vi "Modelo planta H2_V2.vi"() -> ()   [LabVIEW 2022 SP3]
uses:
  <vilib>/Utility/file.llb/Read Delimited Spreadsheet (DBL).vi
panel:
  out "Compresor":bool
  out "stop 2":bool
  in  "stop":bool
  out "masa total P g":dbl format="%#.1f"
  out "H2 generado dia":dbl format="%#.1f"
  in  "Energía acum H2 verde inicio":dbl=527.0
  out "Energía solar diaría":dbl format="%#.1f"
  in  "Producción Solar total inicio":dbl=3421.0
  in  "H2 generado inicio":dbl=202.8
  out "g H2 consumidos por la FC":dbl
  out "H2 consumido en el lab":dbl=182.6 format="%#.1f"
  out "Numeric 9":dbl format="%#.1f"
  out "Energía acum H2 verde":dbl format="%#.1f"
  out "Producción Solar toral":dbl format="%#.1f"
  out "H2 generado Total":dbl format="%#.1f"
  in  "Forzar Comp":bool
  in  "Pot FC":dbl min=0.0 max=5.0 step=0.5
  in  "Forzar FC":bool
  out "Numeric 4":dbl format="%#.4g"
  out "Potència inversor solar":dbl(graph)
  out "masa total G g":dbl format="%#.0f"
  out "P alta":dbl format="%#.1f"
  out "P baja":dbl format="%#.1f"
  out "Numeric 3":dbl format="%#.4g"
  out "Producción FC":dbl format="%#_2g"
  out "Numeric":dbl format="%#.2f"
  out "Pressió tanc baixa":dbl(graph)
  out "Energia solar no utilitzada":dbl(graph)
  out "Producció d'hidrogen":dbl(graph)
  out "g comprimidos":dbl
  in  "Caudal compresor":dbl
  out "P tanq alta (barg)":dbl(graph)
  out "P tanq baja (barg)":dbl(graph)
  in  "Presión ini Tanq baba":dbl=28.0
  in  "Presión ini Tanq alta":dbl=220.0
  in  "Nº electro":u8 max=6 step=1
  in  "Forzar":bool
  out "Energía Solar no usada (kWh)":dbl(graph)
  out "H2 acumulado diario (g)":dbl(graph)
  out "Producción instalan (g/s)":dbl(graph)
  out "Electroli ON":dbl(graph)
  out "Potencia Consumo electroli instan. (kW)":dbl(graph)
  out "Producción diaria (g)":dbl
  out "Producción instalan (g/s)":dbl
  out "Electroli ON":dbl
  in  "Soleado/Nublado":bool=TRUE
  out "Minuto":i32
  in  "tiempo ejecución":u32=1000
  out "Potencia Solar Instanta (kW)":dbl(graph)
  out "Nublado":dbl[](array[numeric])
  out "Soleado":dbl[](array[numeric])
  out "Minuto":i32
  out "min":i32
  out "Hora":i32
  out "current time":timestamp format="%<%H:%M\n%x>T"
  in  "milliseconds to wait":u32=250
  out "Nublado":dbl[](graph)
  out "Soleado":dbl[](graph)
  # "H2 baixa pressió"
  # "H2 alta pressió"
  # "kW"
  # "barg"
  # "Tanc baixa pressió"
  # "Tanc alta pressió"
  # "Electrolizador"
  # "Compressor"
  # "g/s"
  # "barg"
  # "Solar"
  # "Fuel Cell"
  # "kW"
  # "kW"
  # "g"
  # "g"
  # "Elect ON"
  # "Xarxa electrica"
  # "-"
  # "+"
  # "kW de xarxa"
  # "Producció total d'hidrogen"
  # "Producció d'hidrogen diària"
  # "g"
  # "kg"
  # "Producció total d'energia solar"
  # "Energia solar produïda diària"
  # "kWh"
  # "kWh"
  # "Energia acumulada per H2 verd"
  # "Consum de H2 Lab diari"
  # "g"
  # "kWh"
  # "g"
  # "bar"
  # "bar"
  # "kg"
  # "kWh"
  # "kWh"
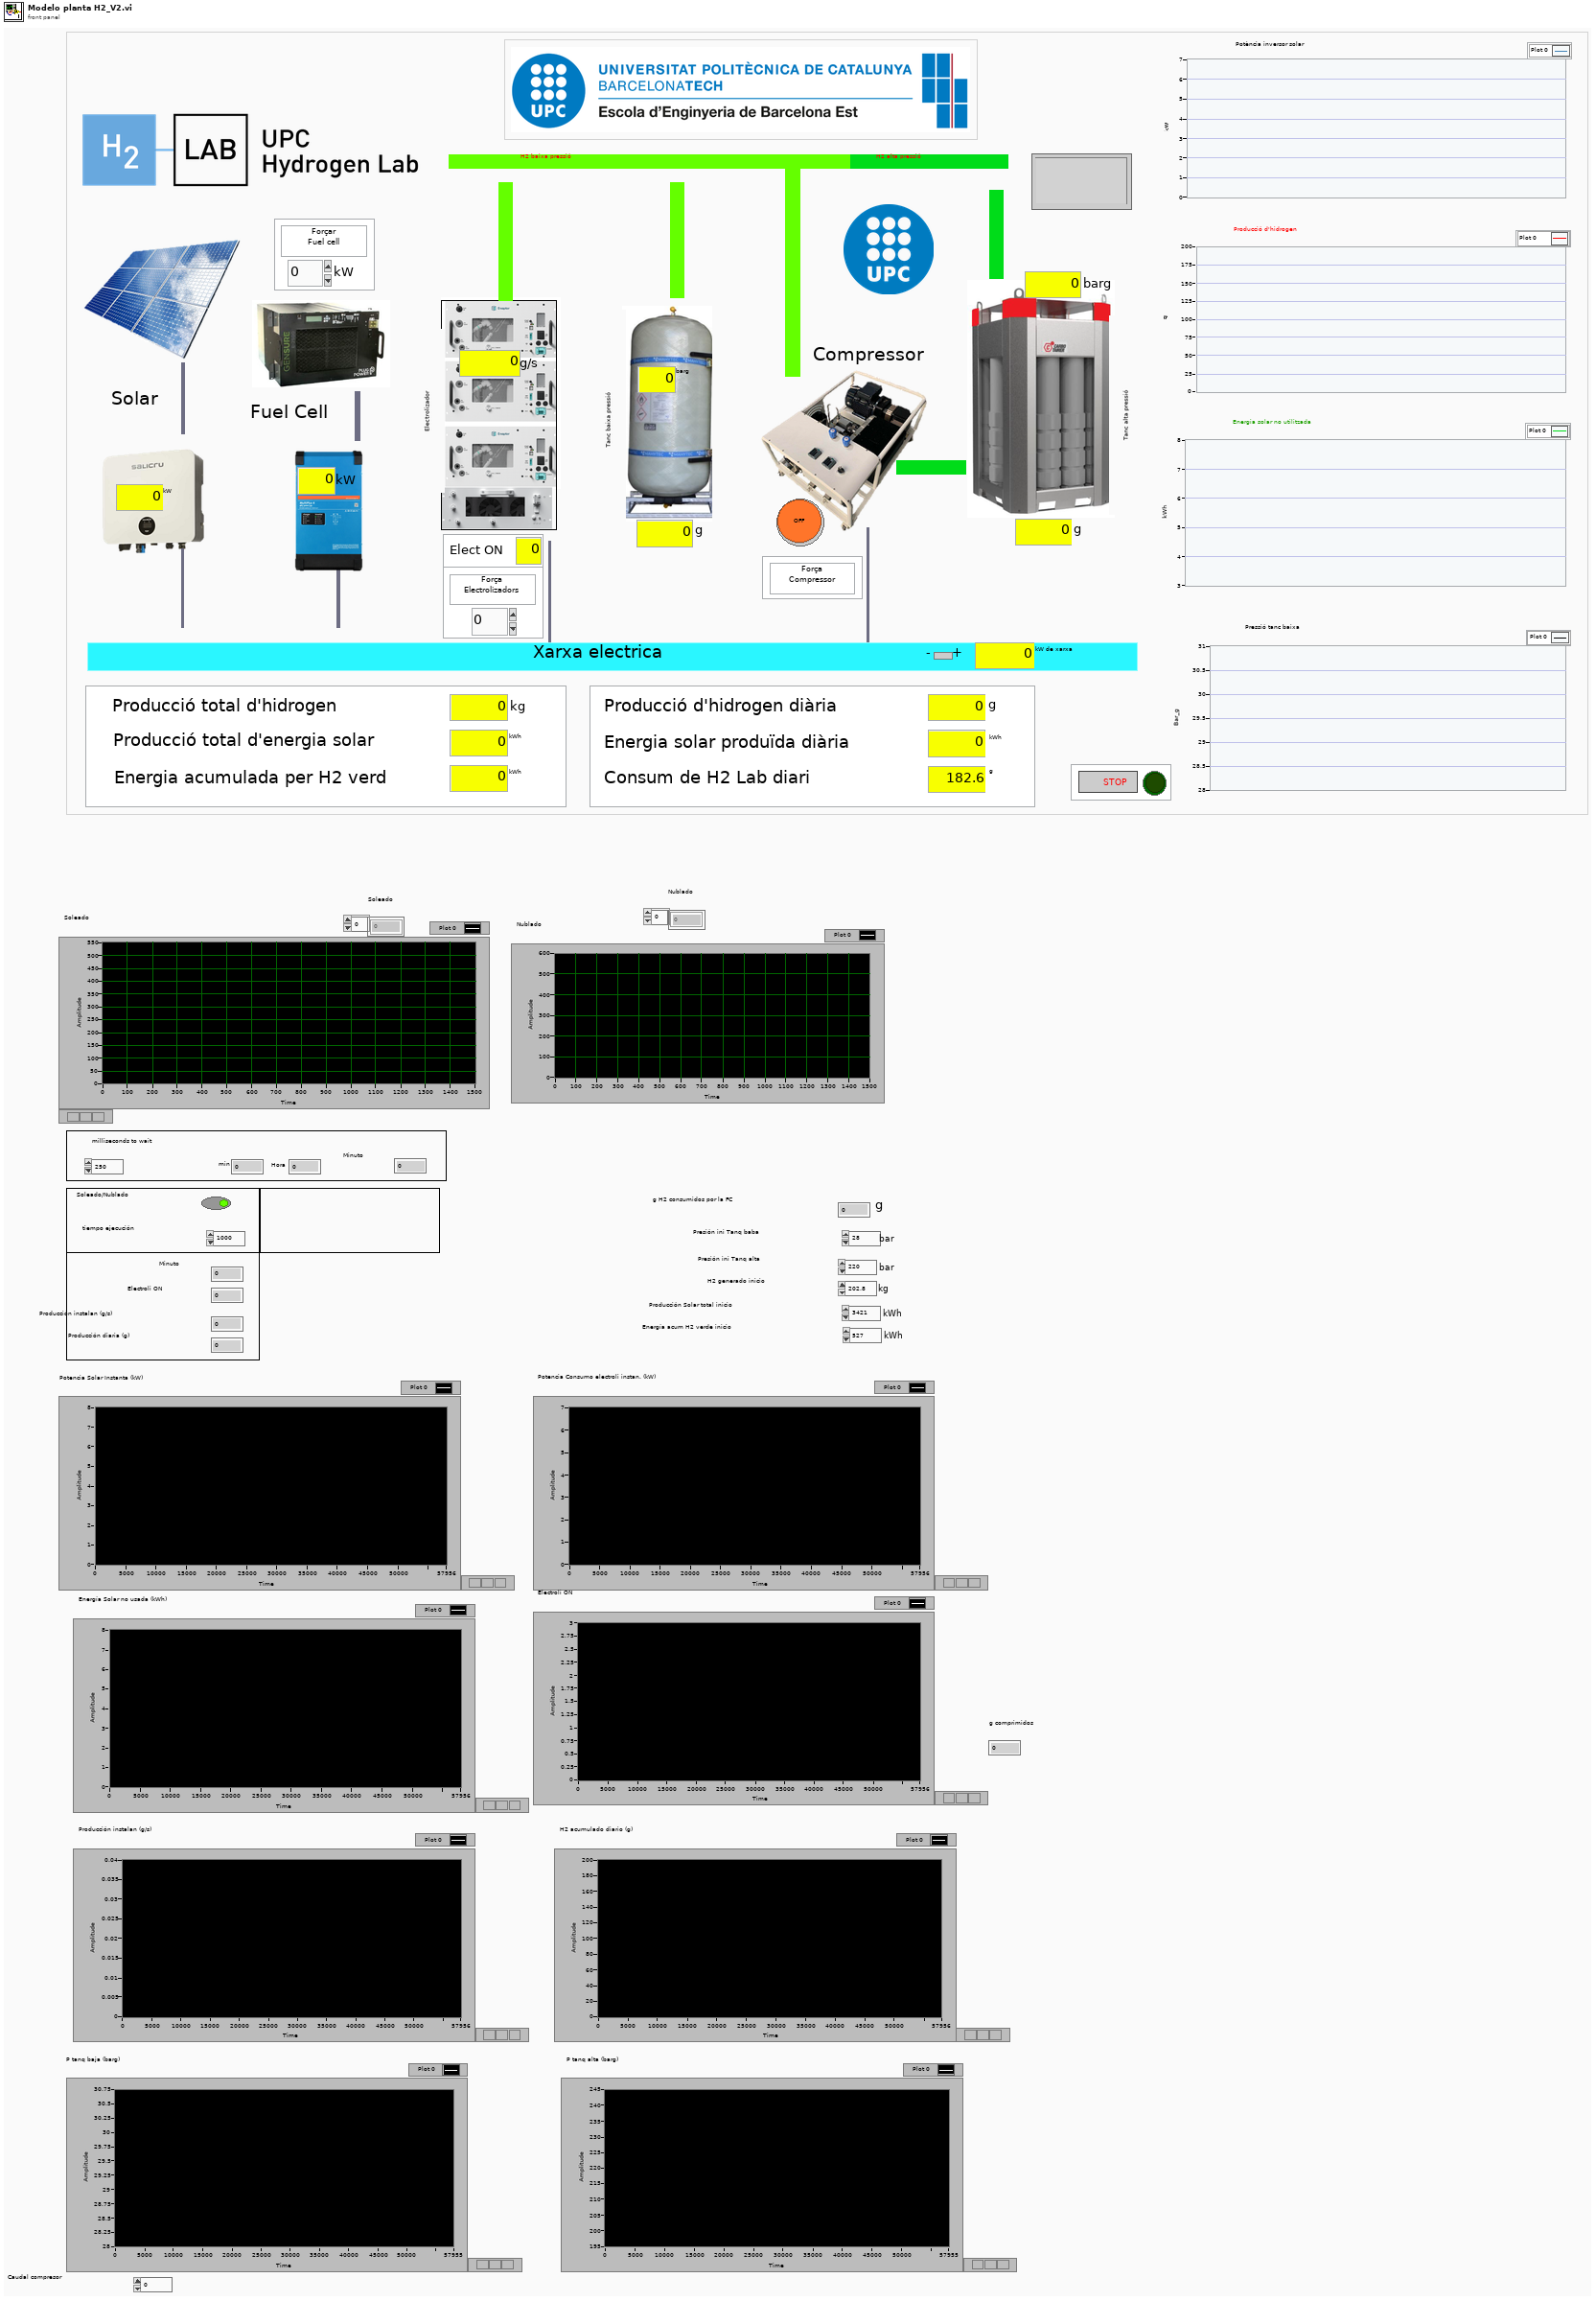
[diagram p1: front panel]
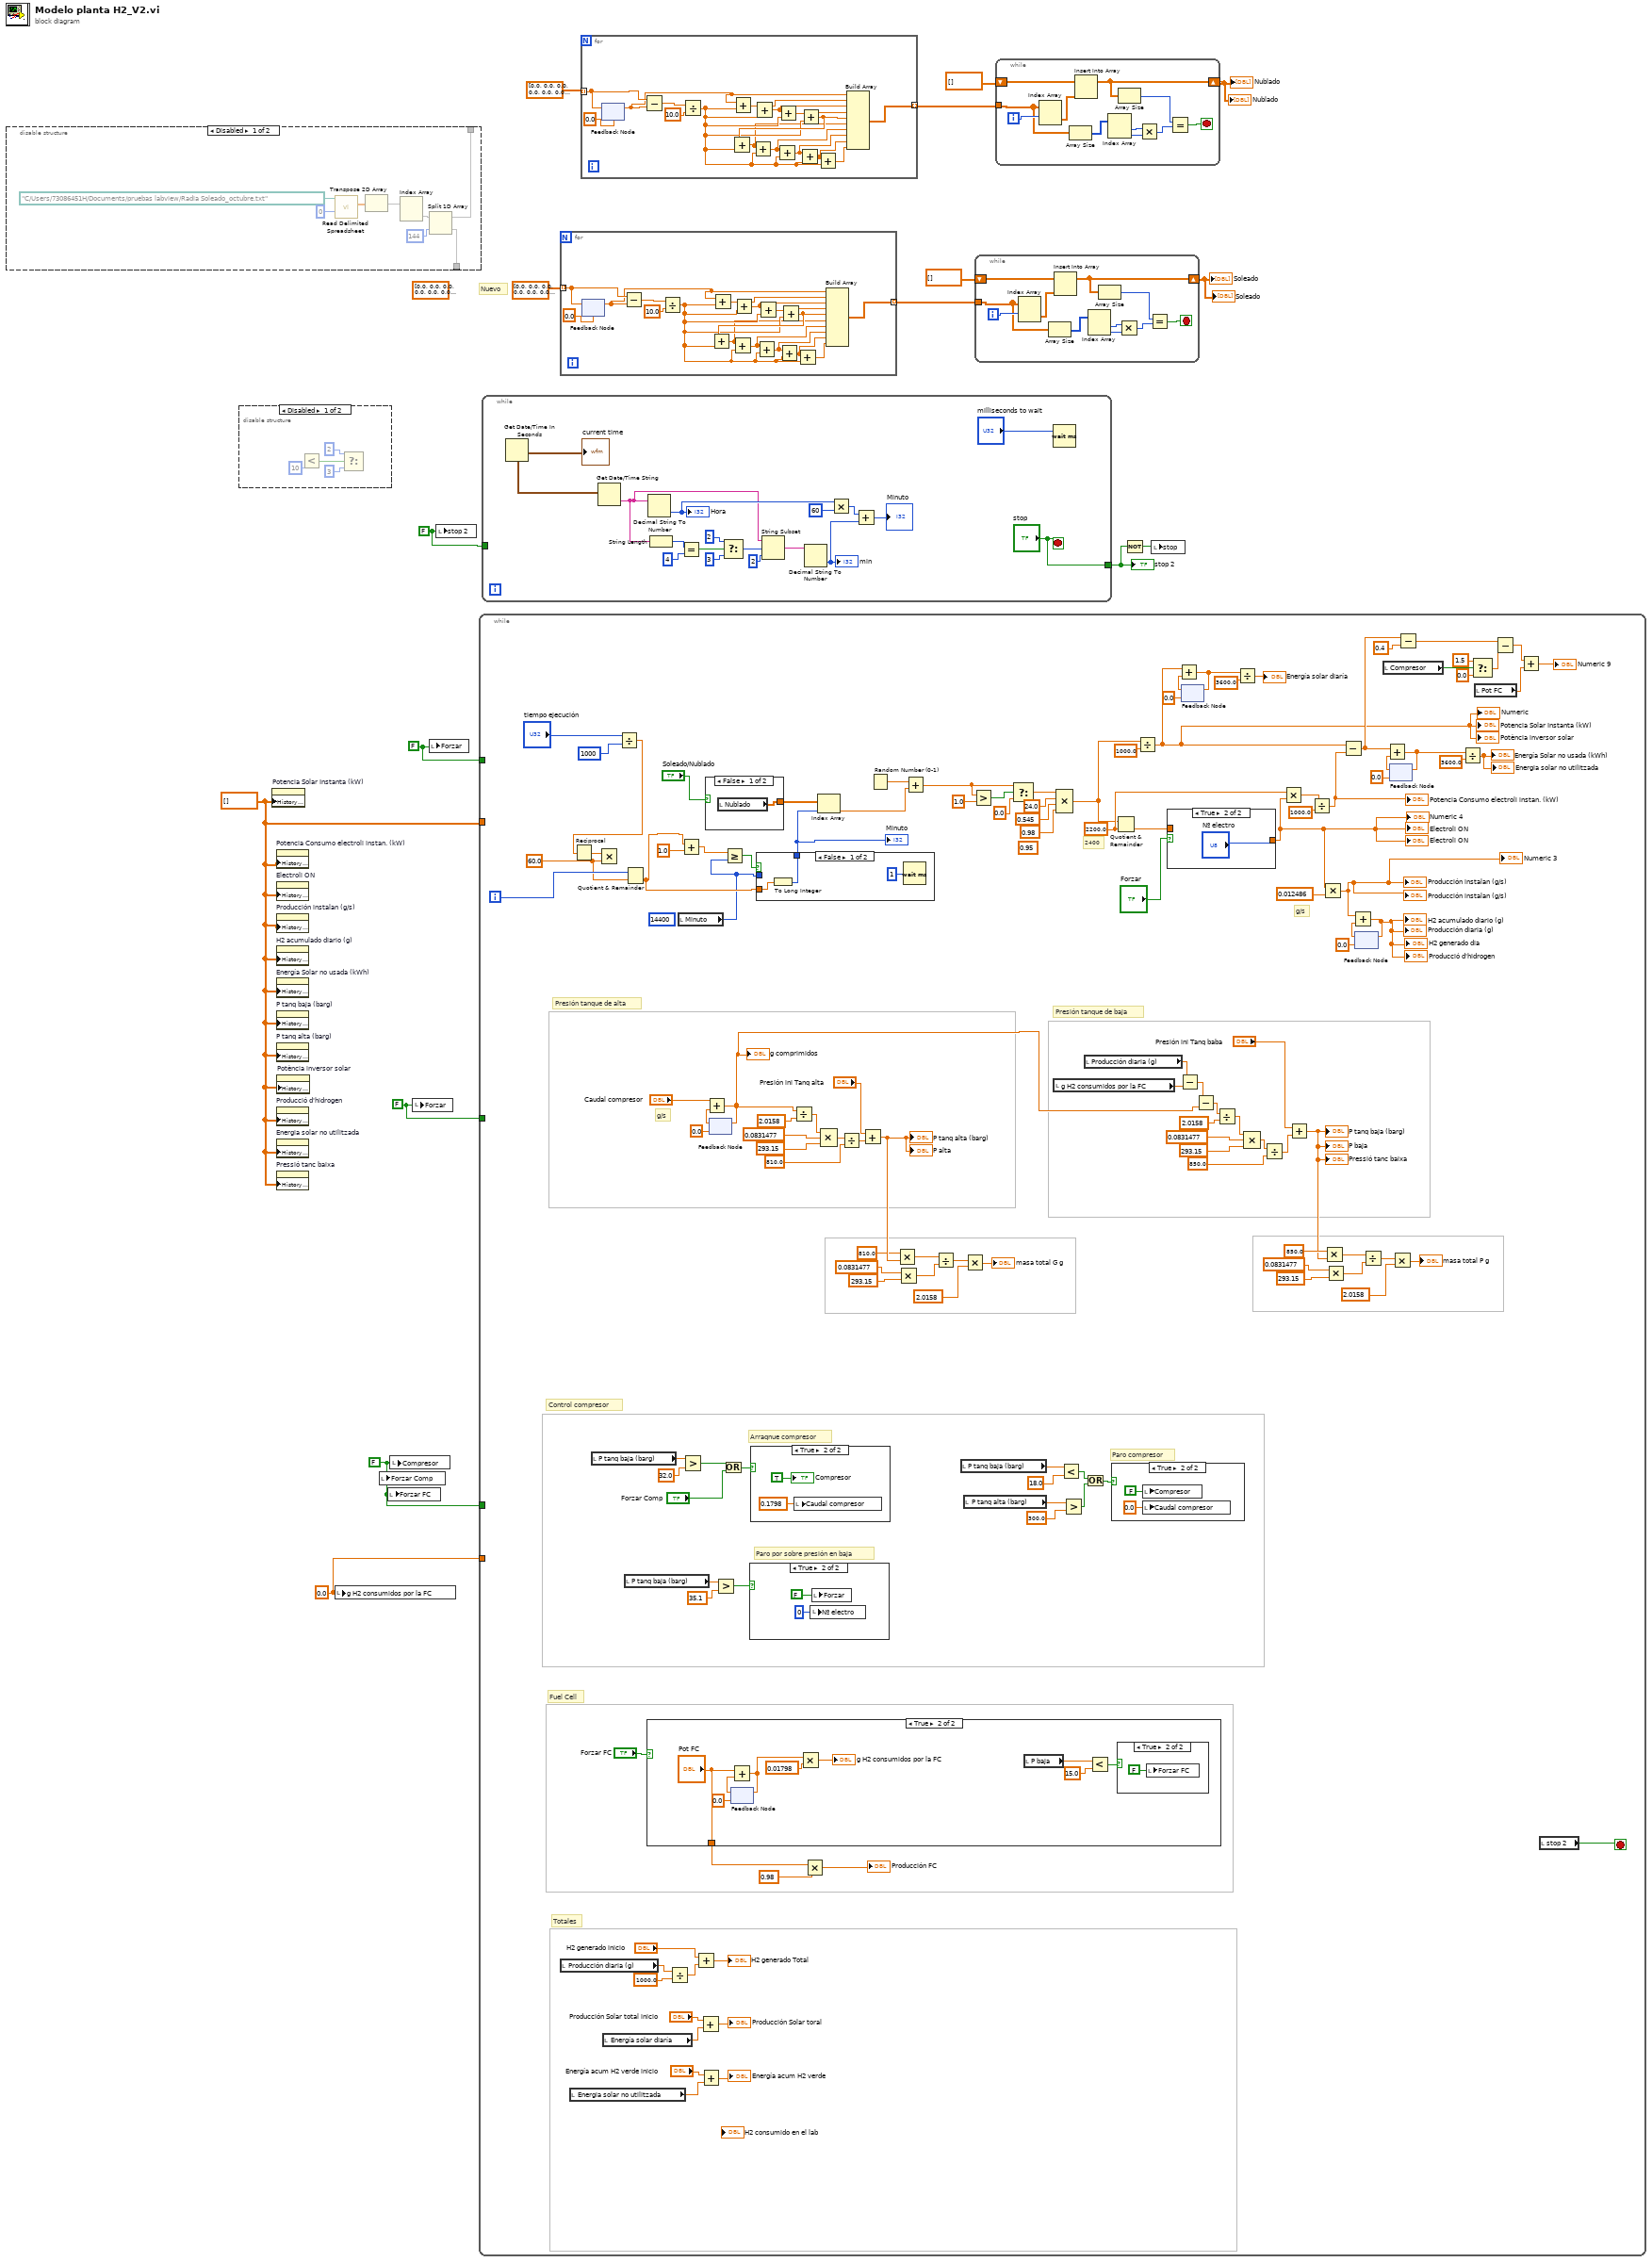
[diagram p0: block diagram]
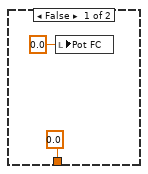
[diagram p4: hidden frame]
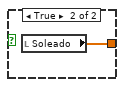
[diagram p10: hidden frame]
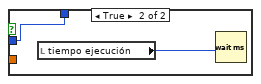
[diagram p11: hidden frame]
diagram:
  w1 = 0.0 ("g H2 consumidos por la FC")
  w3 = FALSE ("stop 2")
  w2 = FALSE ("Compresor")
  (unwired) dbl[] [0.0, 0.0, 0.0, 0.0, 0.0, 0.0, 0.0, 0.0, 0.0, 0.0, 0.0, 0.0, 0.0, 0.0, 0.0, 0.0, 0.0, 0.0, 0.0, 0.0, 0.0, 0.0, 0.0, 0.0, 0.0, 0.0, 0.0, 0.0, 0.0, 0.0, 0.0, 0.0, 0.0, 0.0, 0.0, 0.0, 0.0, 0.0, 0.0, 0.0, 0.0, 0.0, 0.0, 0.0, 0.0, 0.0, 0.0, 20.0, 56.927, 86.927, 116.927, 146.927, 176.927, 206.927, 236.927, 266.927, 296.927, 328.503, 349.407, 367.451, 386.007, 402.123, 418.893, 433.628, 449.442, 458.386, 484.691, 483.049, 496.591, 507.51, 517.195, 522.329, 530.995, 539.123, 538.419, 539.353, 541.627, 542.358, 542.375, 538.101, 543.836, 544.81, 539.48, 533.752, 526.738, 517.297, 506.831, 496.206, 486.59, 477.59, 460.949, 445.951, 431.313, 417.619, 400.78, 383.627, 364.764, 346.383, 329.104, 311.132, 291.528, 271.047, 249.886, 227.664, 206.918, 185.245, 162.013, 141.586, 121.314, 100.961, 79.259, 58.513, 35.892, 22.622, 4.309, 0.0, 0.0, 0.0, 0.0, 0.0, 0.0, 0.0, 0.0, 0.0, 0.0, 0.0, 0.0, 0.0, 0.0, 0.0, 0.0, 0.0, 0.0, 0.0, 0.0, 0.0, 0.0, 0.0, 0.0, 0.0, 0.0, 0.0, 0.0, 0.0] ("first subarray 2")
  w7 = FALSE ("Manual")
  w5 = dbl[] [] ("History Data")
  w9 = FALSE ("stop 2")
  # "Nuevo"
  n1 = disable-structure shown="Disabled" {
    disable-tunnel: [w18 _] -> _
    disable-tunnel: [w17 _] -> _
    frame Disabled {
      n2 = call-poly <vilib>:"Read Delimited Spreadsheet.vi"("file path (dialog if empty)"=path "C:/Users/73086451H/Documents/pruebas labview/Radia Soleado_octubre.txt", "start of read offset (chars.:0)"=0) -> ("all rows"=w23:dbl[][])  [unwired: 8 in, 5 out]
      n3 = Transpose 2D Array(2D array=w23) -> (transposed array=w22:dbl[][])
      n4 = Index Array(array=w22) -> (element=w20:dbl[])  [unwired: 2 in]
      n5 = Split 1D Array(array=w20, index=144) -> (first subarray=w18:dbl[], second subarray=w17:dbl[])
    }
    frame Enabled {
    }
  }
  n6 = disable-structure shown="Disabled" {
    frame Disabled {
      n7 = Less?(y=10) -> (x=w27:i32, x < y?=w29:bool)
      n8 = Select(t=2 ("offset (0)"), s=w29, f=3 ("offset (0)")) -> ()  [unwired: 1 out]
    }
    frame Enabled {
    }
  }
  n9 = property on="Potencia Solar Instanta (kW)" class="WFChart (strict)"("History Data"=w5) -> ()  [unwired: 2 in, 2 out]
  n10 = property on="Potencia Consumo electroli instan. (kW)" class="WFChart (strict)"("History Data"=w5) -> ()  [unwired: 2 in, 2 out]
  n11 = property on="Electroli ON" class="WFChart (strict)"("History Data"=w5) -> ()  [unwired: 2 in, 2 out]
  n12 = property on="Producción instalan (g/s)" class="WFChart (strict)"("History Data"=w5) -> ()  [unwired: 2 in, 2 out]
  n13 = property on="H2 acumulado diario (g)" class="WFChart (strict)"("History Data"=w5) -> ()  [unwired: 2 in, 2 out]
  n14 = property on="Energía Solar no usada (kWh)" class="WFChart (strict)"("History Data"=w5) -> ()  [unwired: 2 in, 2 out]
  n15 = property on="P tanq baja (barg)" class="WFChart (strict)"("History Data"=w5) -> ()  [unwired: 2 in, 2 out]
  n16 = property on="P tanq alta (barg)" class="WFChart (strict)"("History Data"=w5) -> ()  [unwired: 2 in, 2 out]
  n17 = property on="Producció d'hidrogen" class="WFChart (strict)"("History Data"=w5) -> ()  [unwired: 2 in, 2 out]
  n18 = property on="Energia solar no utilitzada" class="WFChart (strict)"("History Data"=w5) -> ()  [unwired: 2 in, 2 out]
  n19 = property on="Pressió tanc baixa" class="WFChart (strict)"("History Data"=w5) -> ()  [unwired: 2 in, 2 out]
  n20 = property on="Potència inversor solar" class="WFChart (strict)"("History Data"=w5) -> ()  [unwired: 2 in, 2 out]
  n21 = local write "g H2 consumidos por la FC"(w1) -> ()
  n22 = local write "Forzar Comp"(w2) -> ()
  n23 = local write "Forzar FC"(w2) -> ()
  n24 = local write "Compresor"(w2) -> ()
  n25 = local write "Forzar"(w7) -> ()
  n26 = local write "Forzar"(w3) -> ()
  n27 = local write "stop 2"(w9) -> ()
  n28 = while {
    tunnel: w5 -> [_]
    tunnel: w7 -> [_]
    tunnel: w2 -> [_]
    tunnel: w3 -> [_]
    tunnel: w1 -> [_]
    i -> [w161]
    stop <- w153 stop-if-true
    (unwired) 0.95 ("f")
    (unwired) 14400 ("Minuto")
    w134 = 2200.0 ("y")
    w139 = 60.0 ("y")
    # "Totales"
    # "Fuel Cell"
    # "Paro por sobre presión en baja"
    # "Paro compresor"
    # "Arraqnue compresor"
    # "g/s"
    # "Control compresor"
    # "Presión tanque de alta"
    # "Presión tanque de baja"
    # "g/s"
    # "2400"
    n29 = local read "Producción diaria (g)"() -> (w60:dbl)
    n30 = local read "Energia solar no utilitzada"() -> (w43:dbl)
    n31 = local read "P tanq baja (barg)"() -> (w116:dbl)
    n32 = local read "Energía solar diaría"() -> (w47:dbl)
    n33 = Divide(x="tiempo ejecución", y=u32 1000) -> (x/y=w150:dbl)
    n34 = Reciprocal(x=w150) -> (1/x=w144:dbl)
    n35 = Multiply(x=w144, y=w139) -> ()  [unwired: 1 out]
    n36 = local read "P tanq baja (barg)"() -> (w104:dbl)
    n37 = Quotient & Remainder(x=w161, y=w139) -> (floor(x/y)=w146:dbl)  [unwired: 1 out]
    n38 = case shown="True" "Forzar FC" {
      tunnel: [0.0 ("Pot FC") "Pot FC"] -> w39
      frame False {
        n39 = local write "Pot FC"(0.0 ("Pot FC")) -> ()
      }
      frame True {
        n40 = feedback #1(0.0) -> (w172:dbl)
        n41 = Add(x="Pot FC", y=w172) -> (x+y=w170:dbl)
        n42 = feedback-in #1(w170) -> ()
        n43 = Multiply(x=w170, y=0.01798) -> (x*y=→"g H2 consumidos por la FC":dbl)
        n44 = local read "P baja"() -> (w167:dbl)
        n45 = Less?(x=w167, y=15.0) -> (x < y?=w165:bool)
        n46 = case shown="True" w165 {
          frame False {
          }
          frame True {
            n47 = local write "Forzar FC"(FALSE ("Forzar FC")) -> ()
          }
        }
      }
    }
    n48 = Divide(x=w60, y=1000.0) -> (x/y=w58:dbl)
    n49 = local read "Minuto"() -> (w76:i32)
    n50 = Add(x=w146, y=1.0) -> (x+y=w147:dbl)
    n51 = Greater?(x=w116, y=32.0) -> (0:w70:bool)
    n52 = Add(x="H2 generado inicio", y=w58) -> (x+y=→"H2 generado Total":dbl)
    n53 = Add(x="Producción Solar total inicio", y=w47) -> (x+y=→"Producción Solar toral":dbl)
    n54 = Add(x="Energía acum H2 verde inicio", y=w43) -> (x+y=→"Energía acum H2 verde":dbl)
    n55 = case shown="False" "Soleado/Nublado" {
      tunnel: [w182 w183] -> w154
      frame False {
        n56 = local read "Nublado"() -> (w182:dbl[])
      }
      frame True {
        n57 = local read "Soleado"() -> (w183:dbl[])
      }
    }
    n58 = feedback #2(0.0) -> (w107:dbl)
    n59 = Add(x="Caudal compresor", y=w107) -> (x+y=w92:dbl)
    "g comprimidos" <- w92
    n60 = feedback-in #2(w92) -> ()
    n61 = Greater?(x=w104, y=35.1) -> (0:w103:bool)
    n62 = Or(x=w70, y="Forzar Comp") -> (x .or. y?=w69:bool)
    n63 = Greater Or Equal?(x=w147, y=w76) -> (x >= y?=w148:bool)
    n64 = case shown="True" w103 {
      frame False {
      }
      frame True {
        n65 = local write "Nº electro"(u8 0 ("Nº electro")) -> ()
        n66 = local write "Forzar"(FALSE ("Manual")) -> ()
      }
    }
    n67 = case shown="True" w69 {
      frame False {
      }
      frame True {
        n68 = local write "Caudal compresor"(0.1798 ("Caudal compresor")) -> ()
        "Compresor" <- TRUE ("Compresor")
      }
    }
    n69 = case shown="False" w148 {
      tunnel: w146 -> [w186 _]
      tunnel: [w185 w187] -> w145
      tunnel: w76 -> [_ w187]
      frame False {
        n70 = To Long Integer(number=w186) -> (32bit integer=w185:i32)
        n71 = Wait (ms)(milliseconds to wait=u32 1) -> ()  [unwired: 1 out]
      }
      frame True {
        n72 = local read "tiempo ejecución"() -> (w188:u32)
        n73 = Wait (ms)(milliseconds to wait=w188) -> ()  [unwired: 1 out]
      }
    }
    "Minuto" <- w145
    n74 = Divide(x=w92, y=2.0158) -> (x/y=w90:dbl)
    n75 = Multiply(x=w39, y=0.98) -> (x*y=→"Producción FC":dbl)
    n76 = Index Array(array=w154, index=w145) -> (element=w159:dbl)
    n77 = Compound Arithmetic op=MULTIPLY(w90, 0.0831477 ("y"), 293.15 ("y")) -> (w119:dbl)
    n78 = Divide(x=w119, y=810.0) -> (x/y=w118:dbl)
    n79 = Add(x="Presión ini Tanq alta", y=w118) -> (x+y=w100:dbl)
    "P tanq alta (barg)" <- w100
    "P alta" <- w100
    n80 = Random Number (0-1)() -> (number: 0 to 1=w160:dbl)
    n81 = Multiply(x=810.0 ("y"), y=w100) -> (x*y=w101:dbl)
    n82 = Multiply(x=0.0831477 ("y"), y=293.15) -> (x*y=w95:dbl)
    n83 = Add(x=w160, y=w159) -> (x+y=w157:dbl)
    n84 = Divide(x=w101, y=w95) -> (x/y=w94:dbl)
    n85 = local read "P tanq baja (barg)"() -> (w113:dbl)
    n86 = Multiply(x=w94, y=2.0158) -> (x*y=→"masa total G g":dbl)
    n87 = local read "P tanq alta (barg)"() -> (w111:dbl)
    n88 = Greater?(x=w157, y=1.0) -> (0:w155:bool)
    n89 = Select(t=w157, s=w155, f=0.0) -> (s? t:f=w143:dbl)
    n90 = local read "g H2 consumidos por la FC"() -> (w61:dbl)
    n91 = Compound Arithmetic op=MULTIPLY(w143, 24.0 ("f"), 0.545 ("f"), 0.98 ("f")) -> (w126:dbl)
    n92 = Less?(x=w113, y=18.0) -> (x < y?=w110:bool)
    n93 = Greater?(x=w111, y=300.0) -> (0:w109:bool)
    n94 = local read "Producción diaria (g)"() -> (w63:dbl)
    n95 = Or(x=w110, y=w109) -> (x .or. y?=w55:bool)
    n96 = case shown="True" w55 {
      frame False {
      }
      frame True {
        n97 = local write "Compresor"(FALSE ("Compresor")) -> ()
        n98 = local write "Caudal compresor"(0.0 ("Caudal compresor")) -> ()
      }
    }
    n99 = Quotient & Remainder(x=w126, y=w134) -> (floor(x/y)=w128:dbl)  [unwired: 1 out]
    n100 = Divide(x=w126, y=1000.0) -> (x/y=w49:dbl)
    "Potencia Solar Instanta (kW)" <- w49
    "Numeric" <- w49
    "Potència inversor solar" <- w49
    n101 = case shown="True" "Forzar" {
      tunnel: w128 -> [w180 _]
      tunnel: [w180 "Nº electro"] -> w79
      frame False {
      }
      frame True {
      }
    }
    "Electroli ON" <- w79
    "Electroli ON" <- w79
    "Numeric 4" <- w79
    n102 = Subtract(x=w63, y=w61) -> (x-y=w62:dbl)
    n103 = feedback #3(0.0) -> (w50:dbl)
    n104 = Add(x=w49, y=w50) -> (x+y=w52:dbl)
    n105 = feedback-in #3(w52) -> ()
    n106 = Subtract(x=w62, y=w92) -> (x-y=w83:dbl)
    n107 = Divide(x=w83, y=2.0158) -> (x/y=w88:dbl)
    n108 = Divide(x=w52, y=3600.0) -> (x/y=→"Energía solar diaría":dbl)
    n109 = Compound Arithmetic op=MULTIPLY(w88, 0.0831477 ("y"), 293.15 ("y")) -> (w86:dbl)
    n110 = Divide(x=w86, y=850.0) -> (x/y=w82:dbl)
    n111 = Multiply(x=w134, y=w79) -> (x*y=w124:dbl)
    n112 = Add(x="Presión ini Tanq baba", y=w82) -> (x+y=w30:dbl)
    "P tanq baja (barg)" <- w30
    "P baja" <- w30
    "Pressió tanc baixa" <- w30
    n113 = Divide(x=w124, y=1000.0) -> (x/y=w123:dbl)
    "Potencia Consumo electroli instan. (kW)" <- w123
    n114 = Multiply(x=w79, y=0.012486) -> (x*y=w102:dbl)
    "Producción instalan (g/s)" <- w102
    "Producción instalan (g/s)" <- w102
    "Numeric 3" <- w102
    n115 = Multiply(x=850.0 ("y"), y=w30) -> (x*y=w32:dbl)
    n116 = Multiply(x=0.0831477 ("y"), y=293.15) -> (x*y=w35:dbl)
    n117 = Subtract(x=w49, y=w123) -> (x-y=w78:dbl)
    n118 = feedback #4(0.0) -> (w136:dbl)
    n119 = Add(x=w102, y=w136) -> (x+y=w42:dbl)
    "Producción diaria (g)" <- w42
    "H2 acumulado diario (g)" <- w42
    "Producció d'hidrogen" <- w42
    "H2 generado dia" <- w42
    n120 = feedback-in #4(w42) -> ()
    n121 = Divide(x=w32, y=w35) -> (x/y=w36:dbl)
    n122 = local read "Compresor"() -> (w75:bool)
    n123 = feedback #5(0.0) -> (w133:dbl)
    n124 = Add(x=w78, y=w133) -> (x+y=w131:dbl)
    n125 = feedback-in #5(w131) -> ()
    n126 = Multiply(x=w36, y=2.0158) -> (x*y=→"masa total P g":dbl)
    n127 = Subtract(x=w78, y=0.4) -> (x-y=w71:dbl)
    n128 = Divide(x=w131, y=3600.0) -> (x/y=→"Energía Solar no usada (kWh)" →"Energia solar no utilitzada":dbl)
    n129 = Select(t=1.5, s=w75, f=0.0 ("t")) -> (s? t:f=w72:dbl)
    n130 = local read "Pot FC"() -> (w64:dbl)
    n131 = Subtract(x=w71, y=w72) -> (x-y=w66:dbl)
    n132 = Add(x=w66, y=w64) -> (x+y=→"Numeric 9":dbl)
    n133 = local read "stop 2"() -> (w153:bool)
  }
  n134 = while {
    tunnel: ["stop"] -> w11
    tunnel: w9 -> [_]
    stop <- "stop" stop-if-true
    n135 = Get Date/Time In Seconds() -> (seconds since 1Jan1904=w204:timestamp)
    "current time" <- w204
    n136 = Get Date/Time String(seconds (now)=w204) -> (time string=w190:string)  [unwired: 2 in, 1 out]
    n137 = Decimal String To Number(string=w190) -> (number=w196:i32)  [unwired: 2 in, 1 out]
    "Hora" <- w196
    n138 = String Length(string=w190) -> (length=w195:i32)
    n139 = Equal?(x=w195, y=4 ("x")) -> (x = y?=w194:bool)
    n140 = Select(t=2 ("offset (0)"), s=w194, f=3 ("offset (0)")) -> (s? t:f=w189:i32)
    n141 = String Subset(string=w190, offset (0)=w189, length (rest)=2 ("length (rest)")) -> (substring=w202:string)
    n142 = Decimal String To Number(string=w202) -> (number=w199:i32)  [unwired: 2 in, 1 out]
    "min" <- w199
    n143 = Multiply(x=w196, y=60) -> (x*y=w200:i32)
    n144 = Add(x=w200, y=w199) -> (x+y=→"Minuto":i32)
    n145 = Wait (ms)(milliseconds to wait="milliseconds to wait") -> ()  [unwired: 1 out]
  }
  "stop 2" <- w11
  n146 = for {
    tunnel: dbl[] [0.0, 0.0, 0.0, 0.0, 0.0, 0.0, 0.0, 0.0, 0.0, 0.0, 0.0, 0.0, 0.0, 0.0, 0.0, 0.0, 0.0, 0.0, 0.0, 0.0, 0.0, 0.0, 0.0, 0.0, 0.0, 0.0, 0.0, 0.0, 0.0, 0.0, 0.0, 0.0, 0.0, 0.0, 0.0, 0.0, 0.0, 0.0, 0.0, 0.0, 0.0, 0.0, 0.0, 20.0, 56.927, 86.927, 116.927, 146.927, 176.927, 206.927, 236.927, 266.927, 296.927, 328.503, 349.407, 367.451, 386.007, 402.123, 418.893, 433.628, 449.442, 458.386, 484.691, 483.049, 496.591, 507.51, 517.195, 522.329, 530.995, 539.123, 538.419, 539.353, 541.627, 542.358, 542.375, 538.101, 543.836, 544.81, 539.48, 533.752, 526.738, 517.297, 506.831, 496.206, 486.59, 477.59, 460.949, 445.951, 431.313, 417.619, 400.78, 383.627, 364.764, 346.383, 329.104, 311.132, 291.528, 271.047, 249.886, 227.664, 206.918, 185.245, 162.013, 141.586, 121.314, 100.961, 79.259, 58.513, 35.892, 22.622, 4.309, 0.0, 0.0, 0.0, 0.0, 0.0, 0.0, 0.0, 0.0, 0.0, 0.0, 0.0, 0.0, 0.0, 0.0, 0.0, 0.0, 0.0, 0.0, 0.0, 0.0, 0.0, 0.0, 0.0, 0.0, 0.0, 0.0, 0.0, 0.0, 0.0, 0.0, 0.0, 0.0, 0.0] ("first subarray 2") -> [w215] mode=indexing
    tunnel: [w206] -> w16 mode=indexing
    n147 = feedback #6(0.0 ("Numeric")) -> (w214:dbl)
    n148 = feedback-in #6(w215) -> ()
    n149 = Subtract(x=w215, y=w214) -> (x-y=w221:dbl)
    n150 = Divide(x=w221, y=10.0) -> (x/y=w212:dbl)
    n151 = Add(x=w214, y=w212) -> (x+y=w219:dbl)
    n152 = Add(x=w219, y=w212) -> (x+y=w218:dbl)
    n153 = Add(x=w218, y=w212) -> (x+y=w217:dbl)
    n154 = Add(x=w217, y=w212) -> (x+y=w213:dbl)
    n155 = Add(x=w213, y=w212) -> (x+y=w211:dbl)
    n156 = Add(x=w211, y=w212) -> (x+y=w210:dbl)
    n157 = Add(x=w210, y=w212) -> (x+y=w209:dbl)
    n158 = Add(x=w209, y=w212) -> (x+y=w208:dbl)
    n159 = Add(x=w208, y=w212) -> (x+y=w207:dbl)
    n160 = Build Array(w214, w219, w218, w217, w213, w211, w210, w209, w208, w207) -> (w206:dbl[])
  }
  n161 = for {
    tunnel: dbl[] [0.0, 0.0, 0.0, 0.0, 0.0, 0.0, 0.0, 0.0, 0.0, 0.0, 0.0, 0.0, 0.0, 0.0, 0.0, 0.0, 0.0, 0.0, 0.0, 0.0, 0.0, 0.0, 0.0, 0.0, 0.0, 0.0, 0.0, 0.0, 0.0, 0.0, 0.0, 0.0, 0.0, 0.0, 0.0, 0.0, 0.0, 0.0, 0.0, 0.0, 0.0, 0.0, 0.0, 0.0, 0.097, 0.644, 9.018, 25.549, 11.436, 10.222, 11.153, 16.868, 19.396, 7.376, 11.219, 30.772, 37.928, 28.59, 54.584, 83.744, 108.269, 149.528, 162.157, 138.144, 142.825, 136.738, 143.591, 145.649, 84.034, 62.325, 50.947, 51.14, 96.329, 117.546, 97.125, 149.949, 165.425, 188.39, 272.904, 193.533, 180.291, 220.605, 152.285, 226.775, 253.296, 221.754, 230.924, 446.071, 568.938, 566.706, 387.063, 259.378, 294.139, 356.528, 346.528, 239.418, 301.85, 175.27, 247.682, 212.497, 136.002, 177.707, 132.82, 136.628, 115.33, 110.149, 168.211, 234.042, 191.933, 152.255, 126.083, 103.301, 76.065, 35.551, 6.041, 4.87, 0.0, 0.0, 0.0, 0.0, 0.0, 0.0, 0.0, 0.0, 0.0, 0.0, 0.0, 0.0, 0.0, 0.0, 0.0, 0.0, 0.0, 0.0, 0.0, 0.0, 0.0, 0.0, 0.0, 0.0, 0.0, 0.0, 0.0, 0.0] ("first subarray") -> [w231] mode=indexing
    tunnel: [w222] -> w12 mode=indexing
    n162 = feedback #7(0.0 ("Numeric")) -> (w230:dbl)
    n163 = feedback-in #7(w231) -> ()
    n164 = Subtract(x=w231, y=w230) -> (x-y=w237:dbl)
    n165 = Divide(x=w237, y=10.0) -> (x/y=w228:dbl)
    n166 = Add(x=w230, y=w228) -> (x+y=w235:dbl)
    n167 = Add(x=w235, y=w228) -> (x+y=w234:dbl)
    n168 = Add(x=w234, y=w228) -> (x+y=w233:dbl)
    n169 = Add(x=w233, y=w228) -> (x+y=w229:dbl)
    n170 = Add(x=w229, y=w228) -> (x+y=w227:dbl)
    n171 = Add(x=w227, y=w228) -> (x+y=w226:dbl)
    n172 = Add(x=w226, y=w228) -> (x+y=w225:dbl)
    n173 = Add(x=w225, y=w228) -> (x+y=w224:dbl)
    n174 = Add(x=w224, y=w228) -> (x+y=w223:dbl)
    n175 = Build Array(w230, w235, w234, w233, w229, w227, w226, w225, w224, w223) -> (w222:dbl[])
  }
  n176 = while {
    tunnel: w16 -> [w245]
    shift-right: [w238] -> w14
    shift-left: dbl[] [] ("deleted portion") -> [w248]
    i -> [w247]
    stop <- w244 stop-if-true
    n177 = Index Array(array=w245, index (row)=w247) -> (element=w246:dbl[])  [unwired: 1 in]
    n178 = Array Size(array=w245) -> (size(s)=w242:i32[])
    n179 = Insert Into Array(array=w248, new element=w246) -> (w238:dbl[])  [unwired: 1 in]
    n180 = Index Array(array=w242) -> (element #1=w241:i32, element #2=w240:i32)  [unwired: 2 in]
    n181 = Array Size(array=w238) -> (size(s)=w243:i32)
    n182 = Multiply(x=w241, y=w240) -> (x*y=w239:i32)
    n183 = Equal?(x=w243, y=w239) -> (x = y?=w244:bool)
  }
  "Soleado" <- w14
  "Soleado" <- w14
  n184 = while {
    tunnel: w12 -> [w256]
    shift-right: [w249] -> w8
    shift-left: dbl[] [] ("deleted portion") -> [w259]
    i -> [w258]
    stop <- w255 stop-if-true
    n185 = Index Array(array=w256, index (row)=w258) -> (element=w257:dbl[])  [unwired: 1 in]
    n186 = Array Size(array=w256) -> (size(s)=w253:i32[])
    n187 = Insert Into Array(array=w259, new element=w257) -> (w249:dbl[])  [unwired: 1 in]
    n188 = Index Array(array=w253) -> (element #1=w252:i32, element #2=w251:i32)  [unwired: 2 in]
    n189 = Array Size(array=w249) -> (size(s)=w254:i32)
    n190 = Multiply(x=w252, y=w251) -> (x*y=w250:i32)
    n191 = Equal?(x=w254, y=w250) -> (x = y?=w255:bool)
  }
  "Nublado" <- w8
  "Nublado" <- w8
  n192 = Not(x=w11) -> (.not. x?=w10:bool)
  n193 = local write "stop"(w10) -> ()
